vi "Dresden R2R Sputter 03.02.2018 IY24.vi"() -> ()   [LabVIEW 2009] (continued)
                                stop <- w23837 stop-if-true
                                n19111 = Greater?(x=w23841, y=50) -> (0:w23835:bool)
                                n19112 = case shown="True" w23835 {
                                frame #0 {
                                }
                                frame #1 {
                                n19113 = local write "Error Message"("Start up process cancelled because\nthere is no enough air pressure.\nPlease check air pressure connections." ("Error Message")) -> ()
                                n19114 = local write "Semi"(TRUE ("Semi")) -> ()
                                }
                                }
                                n19115 = local read "Ch3_Air_press_di"() -> (w23836:bool)
                                n19116 = case shown="True" w23836 {
                                tunnel: [TRUE FALSE] -> w23839
                                frame #0 {
                                }
                                frame #1 {
                                n19117 = Wait Until Next ms Multiple(millisecond multiple=u32 200) -> ()  [unwired: 1 out]
                                }
                                }
                                n19118 = local read "Semi"() -> (w23838:bool)
                                n19119 = Or(x=w23839, y=w23838) -> (x .or. y?=w23837:bool)
                                }
                              }
                              frame #1 {
                              }
                            }
                          }
                          frame #1 {
                            n19120 = local read "Semi"() -> (w23847:bool)
                            n19121 = case shown="False" w23847 {
                              frame #0 {
                                n19122 = Wait Until Next ms Multiple(millisecond multiple=u32 1000) -> ()  [unwired: 1 out]
                                n19123 = local write "Ch3_PV0"(TRUE ("PA0")) -> ()
                                n19124 = local write "Ch3_PA0"(TRUE ("PA0")) -> ()
                              }
                              frame #1 {
                              }
                            }
                          }
                        }
                      }
                      frame #1 {
                      }
                    }
                  }
                  frame #2 {
                    n19125 = local read "Semi"() -> (w23851:bool)
                    n19126 = case shown="False" w23851 {
                      frame #0 {
                        n19127 = stacked-sequence {
                          frame #0 {
                            n19128 = local read "Semi"() -> (w23852:bool)
                            n19129 = case shown="False" w23852 {
                              frame #0 {
                                n19130 = while {
                                i -> [w23859]
                                stop <- w23855 stop-if-true
                                n19131 = Greater?(x=w23859, y=50) -> (0:w23853:bool)
                                n19132 = case shown="True" w23853 {
                                frame #0 {
                                }
                                frame #1 {
                                n19133 = local write "Error Message"("Start up process cancelled because\nchamber door is open.\nPlease close the door." ("Error Message")) -> ()
                                n19134 = local write "Semi"(TRUE ("Semi")) -> ()
                                }
                                }
                                n19135 = local read "Ch3_Ds_di"() -> (w23854:bool)
                                n19136 = case shown="False" w23854 {
                                tunnel: [TRUE FALSE] -> w23857
                                frame #0 {
                                }
                                frame #1 {
                                n19137 = Wait Until Next ms Multiple(millisecond multiple=u32 200) -> ()  [unwired: 1 out]
                                }
                                }
                                n19138 = local read "Semi"() -> (w23856:bool)
                                n19139 = Or(x=w23857, y=w23856) -> (x .or. y?=w23855:bool)
                                }
                              }
                              frame #1 {
                              }
                            }
                          }
                          frame #1 {
                            n19140 = local read "Semi"() -> (w23865:bool)
                            n19141 = case shown="False" w23865 {
                              frame #0 {
                                n19142 = local write "Ch3_PV1"(TRUE ("PA0")) -> ()
                                n19143 = local write "Ch3_PA1"(TRUE ("PA0")) -> ()
                                n19144 = Wait Until Next ms Multiple(millisecond multiple=u32 1000) -> ()  [unwired: 1 out]
                              }
                              frame #1 {
                              }
                            }
                          }
                        }
                      }
                      frame #1 {
                      }
                    }
                  }
                  frame #3 {
                    n19145 = local read "Semi"() -> (w23869:bool)
                    n19146 = case shown="False" w23869 {
                      frame #0 {
                        n19147 = stacked-sequence {
                          frame #0 {
                            n19148 = local read "Semi"() -> (w23870:bool)
                            n19149 = case shown="False" w23870 {
                              frame #0 {
                                n19150 = while {
                                i -> [w23877]
                                stop <- w23873 stop-if-true
                                n19151 = Greater?(x=w23877, y=50) -> (0:w23871:bool)
                                n19152 = case shown="True" w23871 {
                                frame #0 {
                                }
                                frame #1 {
                                n19153 = local write "Error Message"("Start up process cancelled because\nsystem water flow is not enough.\nPlease check main water flow connections." ("Error Message")) -> ()
                                n19154 = local write "Semi"(TRUE ("Semi")) -> ()
                                }
                                }
                                n19155 = local read "Cnt_wfs_di"() -> (w23872:bool)
                                n19156 = case shown="False" w23872 {
                                tunnel: [TRUE FALSE] -> w23875
                                frame #0 {
                                }
                                frame #1 {
                                n19157 = Wait Until Next ms Multiple(millisecond multiple=u32 200) -> ()  [unwired: 1 out]
                                }
                                }
                                n19158 = local read "Semi"() -> (w23874:bool)
                                n19159 = Or(x=w23875, y=w23874) -> (x .or. y?=w23873:bool)
                                }
                              }
                              frame #1 {
                              }
                            }
                          }
                          frame #1 {
                            n19160 = local read "Semi"() -> (w23883:bool)
                            n19161 = case shown="False" w23883 {
                              frame #0 {
                                n19162 = Wait Until Next ms Multiple(millisecond multiple=u32 1000) -> ()  [unwired: 1 out]
                                n19163 = local write "Ch3_PV2"(TRUE ("PA0")) -> ()
                                n19164 = local write "Ch3_PA2"(TRUE ("PA0")) -> ()
                              }
                              frame #1 {
                              }
                            }
                          }
                        }
                      }
                      frame #1 {
                      }
                    }
                  }
                  frame #4 {
                    n19165 = local read "Semi"() -> (w23887:bool)
                    n19166 = case shown="False" w23887 {
                      frame #0 {
                        n19167 = disable-structure shown="Disabled" {
                          frame #0 {
                            n19168 = stacked-sequence {
                              frame #0 {
                                n19169 = local read "Semi"() -> (w23888:bool)
                                n19170 = case shown="False" w23888 {
                                frame #0 {
                                n19171 = local write "Ch3_WFC_do"(TRUE ("Ch1_WFC_do")) -> ()
                                }
                                frame #1 {
                                }
                                }
                              }
                              frame #1 {
                                n19172 = local read "Semi"() -> (w23890:bool)
                                n19173 = case shown="False" w23890 {
                                frame #0 {
                                n19174 = while {
                                i -> [w23897]
                                stop <- w23893 stop-if-true
                                n19175 = Greater?(x=w23897, y=50) -> (0:w23891:bool)
                                n19176 = case shown="True" w23891 {
                                frame #0 {
                                }
                                frame #1 {
                                n19177 = local write "Error Message"("Start up process cancelled because\nchamber water flow is not enough.\nPlease check chamber water \nflow connections." ("Error Message")) -> ()
                                n19178 = local write "Semi"(TRUE ("Semi")) -> ()
                                }
                                }
                                n19179 = local read "Ch3_WFS_di"() -> (w23892:bool)
                                n19180 = case shown="False" w23892 {
                                tunnel: [TRUE FALSE] -> w23895
                                frame #0 {
                                }
                                frame #1 {
                                n19181 = Wait Until Next ms Multiple(millisecond multiple=u32 200) -> ()  [unwired: 1 out]
                                n19182 = local write "Ch3_WFC_do"(TRUE ("Ch1_WFC_do")) -> ()
                                }
                                }
                                n19183 = local read "Semi"() -> (w23894:bool)
                                n19184 = Or(x=w23895, y=w23894) -> (x .or. y?=w23893:bool)
                                }
                                }
                                frame #1 {
                                }
                                }
                              }
                              frame #2 {
                                n19185 = local read "Semi"() -> (w23904:bool)
                                n19186 = case shown="False" w23904 {
                                frame #0 {
                                n19187 = Wait Until Next ms Multiple(millisecond multiple=u32 1000) -> ()  [unwired: 1 out]
                                }
                                frame #1 {
                                }
                                }
                              }
                            }
                          }
                          frame #1 {
                          }
                        }
                      }
                      frame #1 {
                      }
                    }
                  }
                  frame #5 {
                    # "ch2 and ch3 trns gv close check"
                    n19188 = local read "Semi"() -> (w23906:bool)
                    n19189 = case shown="False" w23906 {
                      frame #0 {
                        n19190 = stacked-sequence {
                          frame #0 {
                            # "Her ikiside false olduğunda sinyal alnmaz"
                            n19191 = local read "Semi"() -> (w23907:bool)
                            n19192 = case shown="False" w23907 {
                              frame #0 {
                                n19193 = local write "Ch2_Trns_gv_close_do"(TRUE ("Ch1_WFC_do")) -> ()
                              }
                              frame #1 {
                              }
                            }
                          }
                          frame #1 {
                            n19194 = local read "Semi"() -> (w23909:bool)
                            n19195 = case shown="False" w23909 {
                              frame #0 {
                                n19196 = while {
                                i -> [w23916]
                                stop <- w23912 stop-if-true
                                n19197 = Greater?(x=w23916, y=300) -> (0:w23910:bool)
                                n19198 = case shown="True" w23910 {
                                frame #0 {
                                }
                                frame #1 {
                                n19199 = local write "Error Message"("Start up process cancelled because\nchamber Trns GV between \nCH1 and CH2 not closed.\nPlease check  GV connection." ("Error Message")) -> ()
                                n19200 = local write "Semi"(TRUE ("Semi")) -> ()
                                }
                                }
                                n19201 = local read "Ch2_Trns_gv_close_di"() -> (w23911:bool)
                                n19202 = case shown="False" w23911 {
                                tunnel: [TRUE FALSE] -> w23914
                                frame #0 {
                                }
                                frame #1 {
                                n19203 = Wait Until Next ms Multiple(millisecond multiple=u32 200) -> ()  [unwired: 1 out]
                                n19204 = local write "Ch2_Trns_gv_open_do"(FALSE ("Ch1_Trns_gv_open_do")) -> ()
                                n19205 = local write "Ch2_Trns_gv_close_do"(TRUE ("Ch1_Trns_gv_close_do")) -> ()
                                }
                                }
                                n19206 = local read "Semi"() -> (w23913:bool)
                                n19207 = Or(x=w23914, y=w23913) -> (x .or. y?=w23912:bool)
                                }
                              }
                              frame #1 {
                              }
                            }
                          }
                          frame #2 {
                            n19208 = local read "Semi"() -> (w23924:bool)
                            n19209 = case shown="False" w23924 {
                              frame #0 {
                                n19210 = Wait Until Next ms Multiple(millisecond multiple=u32 1000) -> ()  [unwired: 1 out]
                                n19211 = local write "Ch3_PV4"(TRUE ("PA0")) -> ()
                                n19212 = local write "Ch3_PA4"(TRUE ("PA0")) -> ()
                              }
                              frame #1 {
                              }
                            }
                          }
                        }
                      }
                      frame #1 {
                      }
                    }
                  }
                  frame #6 {
                    # "ch3 and ch4 trns gv close check"
                    n19213 = local read "Semi"() -> (w23928:bool)
                    n19214 = case shown="False" w23928 {
                      frame #0 {
                        n19215 = stacked-sequence {
                          frame #0 {
                            # "Her ikiside false olduğunda sinyal alnmaz"
                            n19216 = local read "Semi"() -> (w23929:bool)
                            n19217 = case shown="False" w23929 {
                              frame #0 {
                                n19218 = local write "Ch3_Trns_gv_close_do"(TRUE ("Ch1_WFC_do")) -> ()
                              }
                              frame #1 {
                              }
                            }
                          }
                          frame #1 {
                            n19219 = local read "Semi"() -> (w23931:bool)
                            n19220 = case shown="False" w23931 {
                              frame #0 {
                                n19221 = while {
                                i -> [w23938]
                                stop <- w23934 stop-if-true
                                n19222 = Greater?(x=w23938, y=300) -> (0:w23932:bool)
                                n19223 = case shown="True" w23932 {
                                frame #0 {
                                }
                                frame #1 {
                                n19224 = local write "Error Message"("Start up process cancelled because\nchamber Trns GV between \nCH3 and CH4 not closed.\nPlease check  GV connection." ("Error Message")) -> ()
                                n19225 = local write "Semi"(TRUE ("Semi")) -> ()
                                }
                                }
                                n19226 = local read "Ch3_Trns_gv_close_di"() -> (w23933:bool)
                                n19227 = case shown="False" w23933 {
                                tunnel: [TRUE FALSE] -> w23936
                                frame #0 {
                                }
                                frame #1 {
                                n19228 = Wait Until Next ms Multiple(millisecond multiple=u32 200) -> ()  [unwired: 1 out]
                                n19229 = local write "Ch3_Trns_gv_open_do"(FALSE ("Ch1_Trns_gv_open_do")) -> ()
                                n19230 = local write "Ch3_Trns_gv_close_do"(TRUE ("Ch1_Trns_gv_close_do")) -> ()
                                }
                                }
                                n19231 = local read "Semi"() -> (w23935:bool)
                                n19232 = Or(x=w23936, y=w23935) -> (x .or. y?=w23934:bool)
                                }
                              }
                              frame #1 {
                              }
                            }
                          }
                          frame #2 {
                            n19233 = local read "Semi"() -> (w23946:bool)
                            n19234 = case shown="False" w23946 {
                              frame #0 {
                                n19235 = Wait Until Next ms Multiple(millisecond multiple=u32 1000) -> ()  [unwired: 1 out]
                                n19236 = local write "Ch3_PV5"(TRUE ("PA0")) -> ()
                                n19237 = local write "Ch3_PA5"(TRUE ("PA0")) -> ()
                              }
                              frame #1 {
                              }
                            }
                          }
                        }
                      }
                      frame #1 {
                      }
                    }
                  }
                }
              }
              frame #1 {
              }
            }
          }
          frame #1 {
            # "ROUTINE CHECK"
            n19238 = local read "Semi"() -> (w23950:bool)
            n19239 = case shown="False" w23950 {
              frame #0 {
                n19240 = local read "Ch3_pressure"() -> (w23952:dbl)
                n19241 = Greater Or Equal?(x=w23952, y=0.9) -> (x >= y?=w23951:bool)
                n19242 = case shown="True" w23951 {
                  frame #0 {
                    # "PUMPING CH3 LOWER THAN 0.9 TORR"
                    n19243 = local read "Semi"() -> (w23954:bool)
                    n19244 = case shown="False" w23954 {
                      frame #0 {
                        n19245 = stacked-sequence {
                          frame #0 {
                            # "Close CH-VBV"
                            n19246 = local read "Semi"() -> (w23955:bool)
                            n19247 = case shown="False" w23955 {
                              frame #0 {
                                n19248 = stacked-sequence {
                                frame #0 {
                                n19249 = local read "Semi"() -> (w23956:bool)
                                n19250 = case shown="False" w23956 {
                                frame #0 {
                                n19251 = while {
                                i -> [w23963]
                                stop <- w23957 stop-if-true
                                n19252 = Greater?(x=w23963, y=50) -> (0:w23961:bool)
                                n19253 = case shown="True" w23961 {
                                frame #0 {
                                }
                                frame #1 {
                                n19254 = local write "Semi"(TRUE ("Semi")) -> ()
                                n19255 = local write "Error Message"("Start up process  cancelled\nbecause  CH-VBV not closed.\nPlease check  CH3-VBV connections." ("Error Message")) -> ()
                                }
                                }
                                n19256 = local read "Ch3_Ch_vbv_di"() -> (w23960:bool)
                                n19257 = case shown="True" w23960 {
                                tunnel: [TRUE FALSE] -> w23959
                                frame #0 {
                                }
                                frame #1 {
                                n19258 = Wait Until Next ms Multiple(millisecond multiple=u32 200) -> ()  [unwired: 1 out]
                                n19259 = local write "Ch3_Ch_vbv_do"(FALSE ("Ch1_Tp_bv_do")) -> ()
                                }
                                }
                                n19260 = local read "Semi"() -> (w23958:bool)
                                n19261 = Or(x=w23959, y=w23958) -> (x .or. y?=w23957:bool)
                                }
                                }
                                frame #1 {
                                }
                                }
                                }
                                frame #1 {
                                n19262 = local read "Semi"() -> (w23970:bool)
                                n19263 = case shown="False" w23970 {
                                frame #0 {
                                n19264 = local write "Ch3_PV6"(TRUE ("P03")) -> ()
                                n19265 = Wait Until Next ms Multiple(millisecond multiple=u32 1000) -> ()  [unwired: 1 out]
                                }
                                frame #1 {
                                }
                                }
                                }
                                }
                              }
                              frame #1 {
                              }
                            }
                          }
                          frame #1 {
                            # "Close PL-VBV"
                            n19266 = local read "Semi"() -> (w23973:bool)
                            n19267 = case shown="False" w23973 {
                              frame #0 {
                                n19268 = stacked-sequence {
                                frame #0 {
                                n19269 = local read "Semi"() -> (w23974:bool)
                                n19270 = case shown="False" w23974 {
                                frame #0 {
                                n19271 = while {
                                i -> [w23981]
                                stop <- w23975 stop-if-true
                                n19272 = Greater?(x=w23981, y=50) -> (0:w23979:bool)
                                n19273 = case shown="True" w23979 {
                                frame #0 {
                                }
                                frame #1 {
                                n19274 = local write "Semi"(TRUE ("Semi")) -> ()
                                n19275 = local write "Error Message"("Start up process  cancelled\nbecause  PL-VBV not closed.\nPlease check PL3-VBV connections." ("Error Message")) -> ()
                                }
                                }
                                n19276 = local read "Ch3_Pl_vbv_di"() -> (w23978:bool)
                                n19277 = case shown="True" w23978 {
                                tunnel: [TRUE FALSE] -> w23977
                                frame #0 {
                                }
                                frame #1 {
                                n19278 = Wait Until Next ms Multiple(millisecond multiple=u32 200) -> ()  [unwired: 1 out]
                                n19279 = local write "Ch3_Pl_vbv_do"(FALSE ("Ch1_Tp_bv_do")) -> ()
                                }
                                }
                                n19280 = local read "Semi"() -> (w23976:bool)
                                n19281 = Or(x=w23977, y=w23976) -> (x .or. y?=w23975:bool)
                                }
                                }
                                frame #1 {
                                }
                                }
                                }
                                frame #1 {
                                n19282 = local read "Semi"() -> (w23988:bool)
                                n19283 = case shown="False" w23988 {
                                frame #0 {
                                n19284 = local write "Ch3_PV7"(TRUE ("P03")) -> ()
                                n19285 = Wait Until Next ms Multiple(millisecond multiple=u32 1000) -> ()  [unwired: 1 out]
                                }
                                frame #1 {
                                }
                                }
                                }
                                }
                              }
                              frame #1 {
                              }
                            }
                          }
                          frame #2 {
                            # "Close CH-ATM"
                            n19286 = local read "Semi"() -> (w23991:bool)
                            n19287 = case shown="False" w23991 {
                              frame #0 {
                                n19288 = stacked-sequence {
                                frame #0 {
                                n19289 = local read "Semi"() -> (w23992:bool)
                                n19290 = case shown="False" w23992 {
                                frame #0 {
                                n19291 = while {
                                i -> [w23999]
                                stop <- w23993 stop-if-true
                                n19292 = Greater?(x=w23999, y=50) -> (0:w23997:bool)
                                n19293 = case shown="True" w23997 {
                                frame #0 {
                                }
                                frame #1 {
                                n19294 = local write "Semi"(TRUE ("Semi")) -> ()
                                n19295 = local write "Error Message"("Start up process  cancelled\nbecause CH-ATM not closed.\nPlease check CH3-ATM connections." ("Error Message")) -> ()
                                }
                                }
                                n19296 = local read "Ch3_Ch_atm_di"() -> (w23996:bool)
                                n19297 = case shown="True" w23996 {
                                tunnel: [TRUE FALSE] -> w23995
                                frame #0 {
                                }
                                frame #1 {
                                n19298 = Wait Until Next ms Multiple(millisecond multiple=u32 200) -> ()  [unwired: 1 out]
                                n19299 = local write "Ch3_Ch_atm_do"(TRUE ("Ch1_Tp_bv_do")) -> ()
                                }
                                }
                                n19300 = local read "Semi"() -> (w23994:bool)
                                n19301 = Or(x=w23995, y=w23994) -> (x .or. y?=w23993:bool)
                                }
                                }
                                frame #1 {
                                }
                                }
                                }
                                frame #1 {
                                n19302 = local read "Semi"() -> (w24006:bool)
                                n19303 = case shown="False" w24006 {
                                frame #0 {
                                n19304 = Wait Until Next ms Multiple(millisecond multiple=u32 1000) -> ()  [unwired: 1 out]
                                n19305 = local write "Ch3_PV8"(TRUE ("P03")) -> ()
                                }
                                frame #1 {
                                }
                                }
                                }
                                }
                              }
                              frame #1 {
                              }
                            }
                          }
                          frame #3 {
                            # "Close PL-ATM"
                            n19306 = local read "Semi"() -> (w24009:bool)
                            n19307 = case shown="False" w24009 {
                              frame #0 {
                                n19308 = stacked-sequence {
                                frame #0 {
                                n19309 = local read "Semi"() -> (w24010:bool)
                                n19310 = case shown="False" w24010 {
                                frame #0 {
                                n19311 = while {
                                i -> [w24017]
                                stop <- w24011 stop-if-true
                                n19312 = Greater?(x=w24017, y=50) -> (0:w24015:bool)
                                n19313 = case shown="True" w24015 {
                                frame #0 {
                                }
                                frame #1 {
                                n19314 = local write "Semi"(TRUE ("Semi")) -> ()
                                n19315 = local write "Error Message"("Start up process  cancelled\nbecause PL-ATM not closed.\nPlease check PL3-ATM connections." ("Error Message")) -> ()
                                }
                                }
                                n19316 = local read "Ch3_Pl_atm_di"() -> (w24014:bool)
                                n19317 = case shown="True" w24014 {
                                tunnel: [TRUE FALSE] -> w24013
                                frame #0 {
                                }
                                frame #1 {
                                n19318 = Wait Until Next ms Multiple(millisecond multiple=u32 200) -> ()  [unwired: 1 out]
                                n19319 = local write "Ch3_Pl_atm_do"(TRUE ("Ch1_Tp_bv_do")) -> ()
                                }
                                }
                                n19320 = local read "Semi"() -> (w24012:bool)
                                n19321 = Or(x=w24013, y=w24012) -> (x .or. y?=w24011:bool)
                                }
                                }
                                frame #1 {
                                }
                                }
                                }
                                frame #1 {
                                n19322 = local read "Semi"() -> (w24024:bool)
                                n19323 = case shown="False" w24024 {
                                frame #0 {
                                n19324 = local write "Ch3_PV9"(TRUE ("P03")) -> ()
                                n19325 = Wait Until Next ms Multiple(millisecond multiple=u32 1000) -> ()  [unwired: 1 out]
                                }
                                frame #1 {
                                }
                                }
                                }
                                }
                              }
                              frame #1 {
                              }
                            }
                          }
                          frame #4 {
                            # "START MP"
                            n19326 = local read "Semi"() -> (w24027:bool)
                            n19327 = case shown="False" w24027 {
                              frame #0 {
                                n19328 = stacked-sequence {
                                frame #0 {
                                n19329 = local read "Semi"() -> (w24028:bool)
                                n19330 = case shown="False" w24028 {
                                frame #0 {
                                n19331 = while {
                                i -> [w24035]
                                stop <- w24029 stop-if-true
                                n19332 = Greater?(x=w24035, y=50) -> (0:w24033:bool)
                                n19333 = case shown="True" w24033 {
                                frame #0 {
                                }
                                frame #1 {
                                n19334 = local write "Semi"(TRUE ("Semi")) -> ()
                                n19335 = local write "Error Message"("Start up process  cancelled\nbecause MP not started.\nPlease check MP3 connections." ("Error Message")) -> ()
                                }
                                }
                                n19336 = local read "Ch3_Mp_di"() -> (w24032:bool)
                                n19337 = case shown="False" w24032 {
                                tunnel: [FALSE TRUE] -> w24031
                                frame #0 {
                                n19338 = Wait Until Next ms Multiple(millisecond multiple=u32 200) -> ()  [unwired: 1 out]
                                n19339 = local write "Ch3_Mp_do"(TRUE ("Ch1_Tp_bv_do")) -> ()
                                }
                                frame #1 {
                                }
                                }
                                n19340 = local read "Semi"() -> (w24030:bool)
                                n19341 = Or(x=w24031, y=w24030) -> (x .or. y?=w24029:bool)
                                }
                                }
                                frame #1 {
                                }
                                }
                                }
                                frame #1 {
                                n19342 = local read "Semi"() -> (w24042:bool)
                                n19343 = case shown="False" w24042 {
                                frame #0 {
                                n19344 = local write "Ch3_PV10"(TRUE ("P03")) -> ()
                                n19345 = Wait Until Next ms Multiple(millisecond multiple=u32 1000) -> ()  [unwired: 1 out]
                                }
                                frame #1 {
                                }
                                }
                                }
                                }
                              }
                              frame #1 {
                              }
                            }
                          }
                          frame #5 {
                            # "CHECK PL-PRESSURE"
                            n19346 = local read "Semi"() -> (w24045:bool)
                            n19347 = case shown="False" w24045 {
                              frame #0 {
                                n19348 = stacked-sequence {
                                frame #0 {
                                n19349 = local read "Semi"() -> (w24046:bool)
                                n19350 = case shown="False" w24046 {
                                frame #0 {
                                n19351 = while {
                                i -> [w24055]
                                stop <- w24050 stop-if-true
                                n19352 = Greater?(x=w24055, y=240) -> (0:w24053:bool)
                                n19353 = case shown="True" w24053 {
                                frame #0 {
                                }
                                frame #1 {
                                n19354 = local write "Semi"(TRUE ("Semi")) -> ()
                                n19355 = local write "Error Message"("Start up process was cancelled.\nPlease check Pipeline \nvacuum connections." ("Error Message")) -> ()
                                }
                                }
                                n19356 = local read "Pl_pg_press_ch3"() -> (w24049:dbl)
                                n19357 = Less?(x=w24049, y=0.9) -> (x < y?=w24047:bool)
                                n19358 = case shown="False" w24047 {
                                tunnel: [FALSE TRUE] -> w24052
                                frame #0 {
                                n19359 = Wait Until Next ms Multiple(millisecond multiple=u32 200) -> ()  [unwired: 1 out]
                                }
                                frame #1 {
                                }
                                }
                                n19360 = local read "Semi"() -> (w24051:bool)
                                n19361 = Or(x=w24052, y=w24051) -> (x .or. y?=w24050:bool)
                                }
                                }
                                frame #1 {
                                }
                                }
                                }
                                frame #1 {
                                n19362 = local read "Semi"() -> (w24061:bool)
                                n19363 = case shown="False" w24061 {
                                frame #0 {
                                n19364 = local write "Ch3_PV11"(TRUE ("P03")) -> ()
                                n19365 = Wait Until Next ms Multiple(millisecond multiple=u32 1000) -> ()  [unwired: 1 out]
                                }
                                frame #1 {
                                }
                                }
                                }
                                }
                              }
                              frame #1 {
                              }
                            }
                          }
                          frame #6 {
                            # "CHECK CH-PRESSURE"
                            n19366 = local read "Semi"() -> (w24064:bool)
                            n19367 = case shown="False" w24064 {
                              frame #0 {
                                n19368 = stacked-sequence {
                                frame #0 {
                                n19369 = local read "Semi"() -> (w24065:bool)
                                n19370 = case shown="False" w24065 {
                                frame #0 {
                                n19371 = while {
                                i -> [w24074]
                                stop <- w24069 stop-if-true
                                n19372 = Greater?(x=w24074, y=50) -> (0:w24072:bool)
                                n19373 = case shown="True" w24072 {
                                frame #0 {
                                }
                                frame #1 {
                                n19374 = local write "Semi"(TRUE ("Semi")) -> ()
                                n19375 = local write "Error Message"("Start up process was cancelled.\nPlease check chamber \nvacuum connections." ("Error Message")) -> ()
                                }
                                }
                                n19376 = local read "Ch3_pressure"() -> (w24068:dbl)
                                n19377 = Less?(x=w24068, y=0.9) -> (x < y?=w24066:bool)
                                n19378 = case shown="False" w24066 {
                                tunnel: [FALSE TRUE] -> w24071
                                frame #0 {
                                n19379 = Wait Until Next ms Multiple(millisecond multiple=u32 200) -> ()  [unwired: 1 out]
                                }
                                frame #1 {
                                }
                                }
                                n19380 = local read "Semi"() -> (w24070:bool)
                                n19381 = Or(x=w24071, y=w24070) -> (x .or. y?=w24069:bool)
                                }
                                }
                                frame #1 {
                                }
                                }
                                }
                                frame #1 {
                                n19382 = local read "Semi"() -> (w24080:bool)
                                n19383 = case shown="False" w24080 {
                                frame #0 {
                                n19384 = local write "Ch3_PV12"(TRUE ("P03")) -> ()
                                n19385 = Wait Until Next ms Multiple(millisecond multiple=u32 1000) -> ()  [unwired: 1 out]
                                }
                                frame #1 {
                                }
                                }
                                }
                                }
                              }
                              frame #1 {
                              }
                            }
                          }
                          frame #7 {
                            # "OPEN TP-BV"
                            n19386 = local read "Semi"() -> (w24083:bool)
                            n19387 = case shown="False" w24083 {
                              frame #0 {
                                n19388 = stacked-sequence {
                                frame #0 {
                                n19389 = local read "Semi"() -> (w24084:bool)
                                n19390 = case shown="False" w24084 {
                                frame #0 {
                                n19391 = while {
                                i -> [w24091]
                                stop <- w24086 stop-if-true
                                n19392 = Greater?(x=w24091, y=50) -> (0:w24089:bool)
                                n19393 = case shown="True" w24089 {
                                frame #0 {
                                }
                                frame #1 {
                                n19394 = local write "Semi"(TRUE ("Semi")) -> ()
                                n19395 = local write "Error Message"("Start up process  cancelled\nbecause  TP-BV not opened.\nPlease check TP-BV3 connections." ("Error Message")) -> ()
                                }
                                }
                                n19396 = local read "Ch3_Tp_bv_di"() -> (w24085:bool)
                                n19397 = case shown="False" w24085 {
                                tunnel: [FALSE TRUE] -> w24088
                                frame #0 {
                                n19398 = Wait Until Next ms Multiple(millisecond multiple=u32 200) -> ()  [unwired: 1 out]
                                n19399 = local write "Ch3_Tp_bv_do"(TRUE ("Ch1_Tp_bv_do")) -> ()
                                }
                                frame #1 {
                                }
                                }
                                n19400 = local read "Semi"() -> (w24087:bool)
                                n19401 = Or(x=w24088, y=w24087) -> (x .or. y?=w24086:bool)
                                }
                                }
                                frame #1 {
                                }
                                }
                                }
                                frame #1 {
                                n19402 = local read "Semi"() -> (w24098:bool)
                                n19403 = case shown="False" w24098 {
                                frame #0 {
                                n19404 = local write "Ch3_PV13"(TRUE ("P03")) -> ()
                                n19405 = Wait Until Next ms Multiple(millisecond multiple=u32 1000) -> ()  [unwired: 1 out]
                                }